vi "Martins HOT interface 120420.vi"() -> ()   [LabVIEW 2011] (continued)
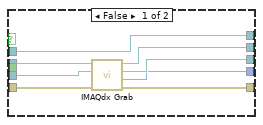
[diagram p6: hidden frame]
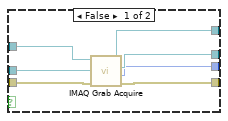
[diagram p7: hidden frame]
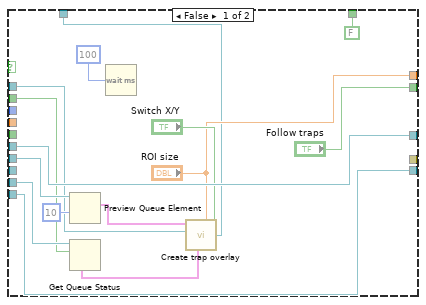
[diagram p9: hidden frame]
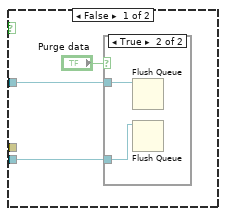
[diagram p11: hidden frame]
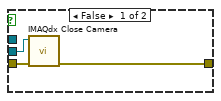
[diagram p16: hidden frame]
              tunnel: w260 -> [_ w344]
              tunnel: w254 -> [_ w343]
              tunnel: w259 -> [_ w342]
              tunnel: w258 -> [_ w341]
              tunnel: [w338 w339] -> w253
              tunnel: w252 -> [w338 w340]
              frame False {
              }
              frame True {
                n77 = call "compute path cluster.vi"("path queue"=w343, "Arrive simultaeously"=w341, "error in (no error)"=w340, "Step length\n(IMAQ pixels)"=w342, "waypoint queue"=w344) -> ("error out"=w339:errorcluster)  [unwired: 2 in]
              }
            }
            n78 = case "Follow path" shown="True" w255 {
              tunnel: w254 -> [_ w289]
              tunnel: w253 -> [_ w290]
              tunnel: w251 -> [_ w292]
              tunnel: w250 -> [_ w291]
              tunnel: w248 -> [_ w288]
              tunnel: w247 -> [w262 w269]
              tunnel: [w262 w268] -> w246
              tunnel: [w261 w263] -> w245
              tunnel: w244 -> [w261 _]
              frame False {
              }
              frame True {
                w283 = TRUE ("Visible")
                n79 = local write "Display path"(FALSE ("Display path")) -> ()
                n80 = Flush Queue "Flush Waypts"(queue=w291, error in (no error)=w290) -> (error out=w282:errorcluster)  [unwired: 2 out]
                n81 = Get Queue Status(queue=w289, error in (no error)=w282) -> (queue out=w286:refnum<queue>, error out=w281:errorcluster, # elements in queue=w285:i32)  [unwired: 1 in, 5 out]
                n82 = property on="Pause" class="Bool (strict)"(error in=w281, "Visible"=w283) -> (error out=w280:errorcluster)  [unwired: 1 in, 1 out]
                n83 = property on="cancel path" class="Bool"(error in=w280, "Visible"=w283) -> (error out=w279:errorcluster)  [unwired: 1 in, 1 out]
                n84 = for {
                  N: w285 -> [_]
                  tunnel: w279 -> [w311]
                  tunnel: w292 -> [w313]
                  tunnel: w286 -> [w309]
                  tunnel: [w309] -> w284
                  tunnel: [FALSE ("Group traps")] -> w264
                  shift-right: [w300] -> w263
                  shift-left: _ -> [w302]
                  tunnel: [w299] -> w278
                  tunnel: [w296] -> w276 mode=indexing
                  tunnel: [w297] -> w272
                  tunnel: [TRUE ("Display path")] -> w270
                  i -> [w297]
                  stop <- w306 stop-if-true
                  n85 = Dequeue Element(queue=w309, timeout in ms (-1)=0, error in (no error)=w311) -> (element=w301:T4, timed out?=w305:bool, error out=w312:errorcluster)  [unwired: 1 out]
                  n86 = while {
                    tunnel: [w330] -> w303
                    tunnel: ["cancel path"] -> w298
                    stop <- w332 stop-if-true
                    n87 = local read "Stop program"() -> (w330:bool)
                    n88 = Wait (ms)(milliseconds to wait="Step time \n(ms)") -> ()  [unwired: 1 out]
                    n89 = Or(x=w330, y="cancel path") -> (x .or. y?=w328:bool)
                    n90 = Implies(1:w328, 2:"Pause") -> (0:w332:bool)
                  }
                  n91 = case shown="True" "Skip step if \ntimed out" {
                    tunnel: w313 -> [w319 w324]
                    tunnel: w312 -> [w318 w322]
                    tunnel: [FALSE ("overflow?") w320] -> w304
                    tunnel: w301 -> [w317 w323]
                    tunnel: [w316 w321] -> w299
                    tunnel: 500 ("timeout in ms (-1)") -> [w315 _]
                    frame False {
                      n92 = Enqueue Element "Enqueue trap pos"(queue=w319, element=w317, timeout in ms (-1)=w315, error in (no error)=w318) -> (error out=w316:errorcluster)  [unwired: 2 out]
                    }
                    frame True {
                      n93 = Lossy Enqueue Element(queue=w324, element=w323, error in (no error)=w322) -> (overflow?=w320:bool, error out=w321:errorcluster)  [unwired: 2 out]
                    }
                  }
                  "Step skipped" <- w304
                  n94 = case shown="False" w303 {
                    tunnel: w302 -> [_ w326]
                    tunnel: w301 -> [w325 _]
                    tunnel: [w325 w326] -> w300
                    frame False {
                    }
                    frame True {
                    }
                  }
                  n95 = Or(x=w298, y=w303) -> (x .or. y?=w308:bool)
                  n96 = Or(x=w308, y=w305) -> (x .or. y?=w306:bool)
                  n97 = Tick Count (ms)() -> (millisecond timer value=w296:u32)
                }
                n98 = local read "Switch X/Y"() -> (w266:bool)
                n99 = call "Trap cluster 2 ROI.vi"("Switch X/Y"=w266, "Trap cluster"=w263, "ROI in"=w288) -> ("ROI out"=w287:T1)
                n100 = local write "Step skipped"(w264) -> ()
                n101 = local write "Display path"(w270) -> ()
                n102 = local write "Create path"(w264) -> ()
                n103 = local write "Group \nTraps"(w264) -> ()
                n104 = property on="Pause" class="Bool (strict)"(error in=w278, "Visible"=w264, "Value"=w264) -> (error out=w277:errorcluster)  [unwired: 1 in, 1 out]
                n105 = property on="cancel path" class="Bool"(error in=w277, "Visible"=w264) -> ()  [unwired: 1 in, 2 out]
                n106 = property on="follow path" class="Bool (strict)"("Value"=w264) -> ()  [unwired: 2 in, 2 out]
                n107 = property on="Image" class="ImageControl"(error in=w269, "ROI"=w287) -> (error out=w268:errorcluster)  [unwired: 1 in, 1 out]
                n108 = Array Max & Min(array=w276) -> (max value=w275:u32, min value=w274:u32)  [unwired: 2 out]
                n109 = Subtract(x=w275, y=w274) -> (x-y=w273:u32)
                n110 = Increment(x=w272) -> (x+1=w267:i32)
                n111 = Divide(x=w273, y=w267) -> (x/y=→"Average step time (ms)":dbl)
                n112 = Flush Queue "Flush Path"(queue=w284) -> ()  [unwired: 1 in, 3 out]
              }
            }
          }
        }
        n113 = case shown="True" "Apply Corrections" {
          frame False {
          }
          frame True {
            n114 = call "Apply Corrections.vi"() -> ()  [unwired: 1 in]
          }
        }
      }
      frame True {
        n115 = property on="Cancel calibration" class="Bool"("Visible"=w346) -> ()  [unwired: 2 in, 2 out]
        n116 = local read "Coordinate mapping \n(IMAQ to SLM)"() -> (w353:T6)
        n117 = flat-sequence {
          tunnel: [w369] -> w359
          tunnel: [w371] -> w358
          tunnel: w354 -> [w369]
          tunnel: w353 -> [w363]
          tunnel: [w360] -> w352
          tunnel: [w363] -> w351
          tunnel: w350 -> [w362]
          tunnel: [w361] -> w348
          tunnel: [w384] -> w357
          tunnel: w359 -> [w384]
          tunnel: w358 -> [w378]
          tunnel: [w380] -> w356
          tunnel: w355 -> [w383]
          tunnel: w352 -> [w382]
          tunnel: w351 -> [w379]
          tunnel: [w376] -> w349
          tunnel: w348 -> [w376]
          tunnel: w357 -> [w439]
          tunnel: w349 -> [w437]
          tunnel: [w436] -> w347
          frame #0 {
            w372 = u32 8 items=["Zoom Tool"=8, "Selection Tool"=0, "Pan Tool"=9, "Point Tool"=1, "Line Tool"=2, "Rectangle Tool"=3, "Rotated Rectangle Tool"=12, "Polyline Tool"=10, "Polygon Tool"=5, "Freehand Tool"=11, "Closed Freehand Tool"=6, "Ellipse Tool"=4, "Annulus Tool"=7] ("Current ROI Tool")
            n118 = Bundle By Name(cluster=w363, "sX"=0.0, "sY"=0.0, "cX"=1.0 ("sX"), "cY"=1.0) -> (w360:T6)
            n119 = local write "Coordinate mapping \n(IMAQ to SLM)"(w360) -> ()
            n120 = property on="ok" class="Bool"("Visible"=TRUE ("ROI Tool Buttons Visibile:Zoom Tool Button Visible")) -> ()  [unwired: 2 in, 2 out]
            n121 = property on="Image" class="ImageControl"("Current ROI Tool"=w372) -> ()  [unwired: 2 in, 2 out]
            n122 = Two Button Dialog(message="Mark the center of the \ndisplayed spot using the \nzoom and the point tool, \nthen click the OK button. \n(Will be repeated three times)", 1:"Cancel" ("F button name (\"Cancel\")"), 2:"Start calibration" ("T button name (\"OK\")")) -> (T button?=w371:bool)
            n123 = property on="Image" class="ImageControl"(error in=w362, "ROI"=T1 {"Global Rectangle"=[100, 100, 394, 354], "Contours"=[{"Contour Type"=0, "ROI Type"=1, "Points"=[100, 100]}]} ("ROI 2")) -> (error out=w361:errorcluster)  [unwired: 1 in, 1 out]
          }
          frame #1 {
            n124 = case shown="True" w378 {
              tunnel: w382 -> [w388 w399]
              tunnel: [w388 w394] -> w381
              tunnel: w383 -> [_ w390]
              tunnel: [TRUE ("Stop program") w389] -> w377
              frame False {
              }
              frame True {
                n125 = for {
                  tunnel: [w426] -> w408 mode=indexing
                  tunnel: [w425] -> w407 mode=indexing
                  tunnel: T4[] [{"X (IMAQ)"=[-64.0], "Y (IMAQ)"=[-64.0], "Z"=[0.0], "I"=[1.0], "Trap number"=[0], "ROI number"=[0], "Number of traps"=1, "Group"=[]}, {"X (IMAQ)"=[64.0], "Y (IMAQ)"=[-64.0], "Z"=[0.0], "I"=[1.0], "Trap number"=[0], "ROI number"=[0], "Number of traps"=1, "Group"=[]}, {"X (IMAQ)"=[-64.0], "Y (IMAQ)"=[64.0], "Z"=[0.0], "I"=[1.0], "Trap number"=[0], "ROI number"=[0], "Number of traps"=0, "Group"=[]}] -> [w423] mode=indexing
                  tunnel: [w420] -> w392 mode=indexing
                  tunnel: [w418] -> w391 mode=indexing
                  tunnel: w390 -> [w422]
                  tunnel: [w417] -> w389
                  stop <- w417 stop-if-true
                  n126 = while {
                    tunnel: [w433] -> w424
                    tunnel: [w429] -> w417
                    stop <- w431 stop-if-true
                    n127 = local read "Stop program"() -> (w430:bool)
                    n128 = Wait (ms)(milliseconds to wait=u32 50) -> ()  [unwired: 1 out]
                    n129 = Or(x=w430, y="Cancel calibration") -> (x .or. y?=w429:bool)
                    n130 = property on="Image" class="ImageControl"() -> ("ROI"=w433:T1)  [unwired: 2 in, 2 out]
                    n131 = Or(x="ok", y=w429) -> (x .or. y?=w431:bool)
                  }
                  n132 = Enqueue Element "Enqueue trap pos"(queue=w422, element=w423) -> ()  [unwired: 2 in, 3 out]
                  n133 = Unbundle By Name(w424) -> ("Global Rectangle"=w427:i32[])  [unwired: 1 out]
                  n134 = Unbundle By Name(w423) -> ("X (IMAQ)"=w421:sgl[], "Y (IMAQ)"=w419:sgl[])
                  n135 = Index Array(array=w421) -> (element=w420:sgl)  [unwired: 1 in]
                  n136 = Index Array(array=w419) -> (element=w418:sgl)  [unwired: 1 in]
                  n137 = Index Array(array=w427) -> (element #1=w426:i32, element #2=w425:i32)  [unwired: 2 in]
                }
                n138 = Index Array(array=w407) -> (element #1=w409:i32, element #2=w410:i32)  [unwired: 2 in]
                n139 = Index Array(array=w408) -> (element #1=w411:i32, element #2=w412:i32)  [unwired: 2 in]
                n140 = Subtract(x=w412, y=w411) -> (x-y=w404:i32)
                n141 = Subtract(x=w410, y=w409) -> (x-y=w402:i32)
                n142 = Absolute Value(x=w402) -> (abs(x)=w401:i32)
                n143 = Absolute Value(x=w404) -> (abs(x)=w403:i32)
                n144 = Less?(x=w403, y=w401) -> (x < y?=w400:bool)
                n145 = case shown="False" w400 {
                  tunnel: w408 -> [w414 w416]
                  tunnel: w407 -> [w413 w415]
                  tunnel: [w413 w416] -> w405
                  tunnel: [w414 w415] -> w406
                  frame False {
                  }
                  frame True {
                  }
                }
                n146 = formula code="cX = (xSLM[1] - xSLM[0]) / (xIMAQ[1] - xIMAQ[0]); \ncY = (ySLM[2] - ySLM[0]) / (yIMAQ[2] - yIMAQ[0]); \n\nsX = xSLM[0] - xIMAQ[0] *cX;\nsY = ySLM[0] - yIMAQ[0] *cY;"("xIMAQ"=w406, "yIMAQ"=w405, "xSLM"=w392, "ySLM"=w391) -> ("cX"=w398:dbl, "cY"=w397:dbl, "sX"=w396:dbl, "sY"=w395:dbl)
                n147 = property on="Switch X/Y" class="Bool (strict)"("Value"=w400) -> ()  [unwired: 2 in, 2 out]
                n148 = Bundle By Name(cluster=w399, "cX"=w398, "cY"=w397, "sX"=w396, "sY"=w395) -> (w394:T6)
              }
            }
            n149 = case "Calibration canceled?" shown="True" w377 {
              tunnel: w381 -> [w385 _]
              tunnel: [w385 w386] -> w380
              tunnel: w379 -> [_ w386]
              frame False {
              }
              frame True {
              }
            }
          }
          frame #2 {
            w435 = FALSE ("ROI Tool Buttons Visibile:Zoom Tool Button Visible")
            w438 = u32 1 items=["Zoom Tool"=8, "Selection Tool"=0, "Pan Tool"=9, "Point Tool"=1, "Line Tool"=2, "Rectangle Tool"=3, "Rotated Rectangle Tool"=12, "Polyline Tool"=10, "Polygon Tool"=5, "Freehand Tool"=11, "Closed Freehand Tool"=6, "Ellipse Tool"=4, "Annulus Tool"=7] ("Current ROI Tool")
            n150 = property on="Image" class="ImageControl"("Current ROI Tool"=w438, "Point Tool Button Visibile"=w435) -> ()  [unwired: 2 in, 2 out]
            n151 = property on="Image" class="ImageControl"(error in=w437, "ROI"=w439) -> (error out=w436:errorcluster)  [unwired: 1 in, 1 out]
            n152 = property on="Cancel" class="Bool"("Visible"=w435) -> ()  [unwired: 2 in, 2 out]
            n153 = property on="ok" class="Bool"("Visible"=w435) -> ()  [unwired: 2 in, 2 out]
          }
        }
        n154 = local write "Coordinate mapping \n(IMAQ to SLM)"(w356) -> ()
      }
    }
  }
  n155 = while "User input and events loop" {
    tunnel: w55 -> [w458]
    tunnel: w15 -> [w447]
    tunnel: w16 -> [w446]
    tunnel: w17 -> [w445]
    tunnel: [w444] -> w31
    tunnel: w30 -> [w443]
    tunnel: [w442] -> w29
    tunnel: w3 -> [w440]
    stop <- w450 stop-if-true
    w455 = u32 8 items=["Zoom Tool"=8, "Selection Tool"=0, "Pan Tool"=9, "Point Tool"=1, "Line Tool"=2, "Rectangle Tool"=3, "Rotated Rectangle Tool"=12, "Polyline Tool"=10, "Polygon Tool"=5, "Freehand Tool"=11, "Closed Freehand Tool"=6, "Ellipse Tool"=4, "Annulus Tool"=7] ("Current ROI Tool")
    w452 = T10 [enum."LCONTROL"] items=["0", "1", "2", "3", "4", "5", "6", "7", "8", "9", "A", "B", "C", "D", "E", "F", "G", "H", "I", "J", "K", "L", "M", "N", "O", "P", "Q", "R", "S", "T", "U", "V", "W", "X", "Y", "Z", "F1", "F2", "F3", "F4", "F5", "F6", "F7", "F8", "F9", "F10", "F11", "F12", "F13", "F14", "F15", "ADD", "BACK", "BACKSLASH", "CAPITAL", "COMMA", "DECIMAL", "DELETE", "DIVIDE", "DOWN", "END", "EQUALS", "ESCAPE", "GRAVE (`)", "HOME", "INSERT", "LBRACKET", "LCONTROL", "LEFT", "L ALT", "LSHIFT", "LWIN", "MINUS", "MULTIPLY", "NEXT", "NUMLOCK", "NUMPAD_0", "NUMPAD_1", "NUMPAD_2", "NUMPAD_3", "NUMPAD_4", "NUMPAD_5", "NUMPAD_6", "NUMPAD_7", "NUMPAD_8", "NUMPAD_9", "PAUSE", "PERIOD", "PRIOR (PG UP)", "RBRACKET", "RCONTROL", "RETURN", "RIGHT", "R ALT", "RSHIFT", "RWIN", "SCROLL", "SEMICOLON", "SLASH", "SPACE", "SUBTRACT", "TAB", "UP", "ENTER (num pad)", "' (quote)"] ("keys pressed")
    n156 = call-poly <vilib>:"Acquire Input Data.vi"("device ID"=w458, "error in (no error)"=w443) -> ("device ID"=w444:refnum<k1>, "keys pressed"=w451:T10, "error out"=w442:errorcluster)  [unwired: 15 out]
    n157 = property on="Image" class="ImageControl"() -> ("Current ROI Tool"=w454:u32)  [unwired: 2 in, 2 out]
    n158 = Equal?(x=w451, y=w452) -> (x = y?=w453:bool[])
    n159 = Not Equal?(x=w454, y=w455) -> (x != y?=w456:bool)
    n160 = Or Array Elements(Boolean array=w453) -> (logical OR=w457:bool)
    n161 = case shown="True" w456 {
      tunnel: w457 -> [_ w492]
      frame False {
      }
      frame True {
        n162 = case shown="False" w492 {
          frame False {
            w493 = u32 0 items=["Zoom Tool"=8, "Selection Tool"=0, "Pan Tool"=9, "Point Tool"=1, "Line Tool"=2, "Rectangle Tool"=3, "Rotated Rectangle Tool"=12, "Polyline Tool"=10, "Polygon Tool"=5, "Freehand Tool"=11, "Closed Freehand Tool"=6, "Ellipse Tool"=4, "Annulus Tool"=7] ("Current ROI Tool")
            n163 = property on="Image" class="ImageControl"("Current ROI Tool"=w493) -> ()  [unwired: 2 in, 2 out]
          }
          frame True {
            w494 = u32 1 items=["Zoom Tool"=8, "Selection Tool"=0, "Pan Tool"=9, "Point Tool"=1, "Line Tool"=2, "Rectangle Tool"=3, "Rotated Rectangle Tool"=12, "Polyline Tool"=10, "Polygon Tool"=5, "Freehand Tool"=11, "Closed Freehand Tool"=6, "Ellipse Tool"=4, "Annulus Tool"=7] ("Current ROI Tool")
            n164 = property on="Image" class="ImageControl"("Current ROI Tool"=w494) -> ()  [unwired: 2 in, 2 out]
          }
        }
      }
    }
    n165 = Wait (ms)(milliseconds to wait=u32 50) -> ()  [unwired: 1 out]
    n166 = case shown="False" "View Licence" {
      frame False {
      }
      frame True {
        n167 = call "View license.vi"() -> ()  [unwired: 1 in]
      }
    }
    n168 = event shown="[1] \"Display hologram\nand computed \nimage plane\": Value Change" {
      selector: _ -> [_ _ _ _ _ _ _ _ _]
      dyn-events: _ -> [_ _ _ _ _ _ _ _ _]
      timeout: 0 -> [_ _ _ _ _ _ _ _ _]
      tunnel: w447 -> [_ _ w469 _ _ _ _ _ _]
      tunnel: w446 -> [_ _ w468 _ _ _ _ _ _]
      tunnel: w445 -> [_ _ w472 _ _ _ _ _ _]
      tunnel: w440 -> [_ _ _ _ _ _ w484 _ _]
      event Timeout {
        n169 = event-data() -> ()  [unwired: 1 in, 2 out]
      }
      event "Display hologram\nand computed \nimage plane": Value Change {
        n170 = event-data() -> ("NewVal"=w460:bool)  [unwired: 1 in, 4 out]
        n171 = property on="Current trap pos" class="Clust (strict)"("Visible"=w460) -> ()  [unwired: 2 in, 2 out]
        n172 = property on="Displayed Hologram" class="IntGraph (strict)"("Visible"=w460) -> ()  [unwired: 2 in, 2 out]
        n173 = property on="Calculated image plane" class="IntGraph (strict)"("Visible"=w460) -> ()  [unwired: 2 in, 2 out]
        n174 = property on="Property Node" class="VI"() -> ("Front Panel.WinBounds"=w467:T11)  [unwired: 2 in, 2 out]
        n175 = Unbundle By Name(w467) -> ("right"=w466:i16, "left"=w465:i16)
        n176 = Subtract(x=w466, y=w465) -> (x-y=w464:i16)
        n177 = Select(t=i16 500 ("x-y"), s=w460, f=i16 196 ("x-y")) -> (s? t:f=w459:i16)
        n178 = Subtract(x=w464, y=w459) -> (x-y=w463:i16)
        n179 = property on="Splitter" class="Splitter"("Position"=w463) -> ()  [unwired: 2 in, 2 out]
      }
      event "Create path": Value Change {
        n180 = event-data() -> ()  [unwired: 1 in, 5 out]
        n181 = property on="follow path" class="Bool (strict)"("Value"=FALSE) -> ()  [unwired: 2 in, 2 out]
        n182 = Flush Queue "Flush path \nwaypt queue"(queue=w468) -> ()  [unwired: 1 in, 3 out]
        n183 = Preview Queue Element(queue=w469) -> (element=w470:T4, error out=w473:errorcluster)  [unwired: 2 in, 2 out]
        n184 = Flush Queue "Flush path queue"(queue=w472) -> (queue out=w471:refnum<queue>)  [unwired: 1 in, 2 out]
        n185 = Enqueue Element "Enqueue current \ntrap pos in path"(queue=w471, element=w470) -> ()  [unwired: 2 in, 3 out]
        n186 = Enqueue Element "Enqueue current \ntrap pos in path \nwaypts"(queue=w468, element=w470, error in (no error)=w473) -> ()  [unwired: 1 in, 3 out]
      }
      event "cancel path": Value Change {
        n187 = event-data() -> ()  [unwired: 1 in, 5 out]
        n188 = local write "Create path"(FALSE ("Visible")) -> ()
      }
      event "Image", "Group \nTraps", "Z", "I", "Coordinate mapping \n(IMAQ to SLM)": Mouse Down {
        w476 = FALSE ("Edit trap cluster")
        n189 = event-data() -> ()  [unwired: 1 in, 7 out]
        n190 = local write "Updating trap cluster"(TRUE ("Update trap positions")) -> ()
        n191 = local write "Edit trap cluster"(w476) -> ()
        n192 = call <vilib>:"Application Directory.vi"() -> ("Application Directory"=w477:path)
        n193 = Build Path(base path=w477, name or relative path="Sub VIs\\Edit trap cluster.vi") -> (appended path=w480:path)
        n194 = Open VI Reference(vi path=w480) -> (vi reference=w479:refnum<vi>)  [unwired: 5 in, 1 out]
        n195 = property class="VI"(reference=w479, "Front Panel.Open"=w476) -> ()  [unwired: 1 in, 2 out]
      }
      event "Group \nTraps", "Z", "I", "Image", "Coordinate mapping \n(IMAQ to SLM)": Mouse Up {
        n196 = event-data() -> ()  [unwired: 1 in, 7 out]
        n197 = flat-sequence {
          frame #0 {
            n198 = Wait (ms)(milliseconds to wait=u32 100) -> ()  [unwired: 1 out]
          }
          frame #1 {
            n199 = local write "Updating trap cluster"(FALSE ("Update trap positions")) -> ()
          }
        }
      }
      event "Video tracking": Value Change {
        n200 = event-data() -> ()  [unwired: 1 in, 5 out]
        n201 = for {
          tunnel: w484 -> [w485] mode=indexing
          n202 = call "IMAQ Clear Overlay"("Image"=w485) -> ()  [unwired: 9 in, 2 out]
        }
      }
      event "Display data": Value Change {
        n203 = event-data() -> ("NewVal"=w487:bool)  [unwired: 1 in, 4 out]
        n204 = call <vilib>:"Application Directory.vi"() -> ("Application Directory"=w486:path)
        n205 = Build Path(base path=w486, name or relative path="Sub VIs\\Display Cetroids (SubVI).vi") -> (appended path=w490:path)
        n206 = Open VI Reference(vi path=w490) -> (vi reference=w489:refnum<vi>)  [unwired: 5 in, 1 out]
        n207 = property class="VI"(reference=w489, "Front Panel.Open"=w487) -> ()  [unwired: 1 in, 2 out]
      }
      event "Edit trap cluster": Value Change {
        n208 = event-data() -> ("NewVal"=w491:bool)  [unwired: 1 in, 4 out]
        n209 = local write "Updating trap cluster"(w491) -> ()
      }
    }
    n210 = local read "Stop program"() -> (w450:bool)
  }
  n211 = disable-structure shown="Disabled" {
    disable-tunnel: [w511 _] -> w54
    disable-tunnel: [w510 _] -> w53
    disable-tunnel: w52 -> [w509 _]
    disable-tunnel: w50 -> [w508 _]
    disable-tunnel: w47 -> [w507 _]
    disable-tunnel: [w506 _] -> w45
    disable-tunnel: [w505 _] -> w44
    disable-tunnel: [w504 _] -> w43
    disable-tunnel: w22 -> [w503 _]
    disable-tunnel: w21 -> [w502 _]
    disable-tunnel: w20 -> [w501 _]
    disable-tunnel: w19 -> [w500 _]
    disable-tunnel: w18 -> [w499 _]
    disable-tunnel: w17 -> [w498 _]
    disable-tunnel: w15 -> [w497 _]
    disable-tunnel: w5 -> [w496 _]
    disable-tunnel: w4 -> [w495 _]
    frame Disabled {
      n212 = while "Image acquisition loop" {
        tunnel: w499 -> [w527]
        tunnel: w495 -> [w551]
        tunnel: w500 -> [w550]
        tunnel: [w523] -> w511
        tunnel: [w549] -> w510
        tunnel: w509 -> [w540]
        tunnel: w508 -> [w547]
        shift-right: [w546] -> _
        shift-left: _ -> [w545]
        tunnel: w507 -> [w544]
        shift-right: [w543] -> _
        shift-left: _ -> [w542]
        tunnel: [w540] -> w506
        tunnel: [w519] -> w505
        tunnel: [w539] -> w504
        tunnel: w503 -> [w538]
        tunnel: w501 -> [w537]
        tunnel: w497 -> [w536]
        tunnel: w498 -> [w535]
        tunnel: w502 -> [w533]
        tunnel: w496 -> [w522]
        i -> [w525]
        stop <- w548 stop-if-true
        n213 = case shown="True" w527 {
          tunnel: w551 -> [w577 w591]
          tunnel: w550 -> [w576 w590]
          tunnel: [w576 w589] -> w521
          tunnel: [w575 w588] -> w549
          tunnel: [w577 w587] -> w515
          tunnel: [w578 w586] -> w539
          tunnel: w538 -> [w578 w585]
          tunnel: w537 -> [_ w584]
          tunnel: w533 -> [w575 w583]
          tunnel: [_ w582] -> w532
          tunnel: w522 -> [_ w581]
          tunnel: w525 -> [_ w580]
          tunnel: "Video tracking" -> [_ w579]
          frame False {
          }
          frame True {
            n214 = case shown="True" w584 {
              tunnel: w591 -> [w599 w610]
              tunnel: [w597 w609] -> w589
              tunnel: [w596 w608] -> w588
              tunnel: w590 -> [w597 w607]
              tunnel: [w598 w606] -> w587
              tunnel: [w593 w605] -> w582
              tunnel: [w595 w604] -> w586
              tunnel: w585 -> [w594 w604]
              tunnel: w583 -> [w592 w603]
              tunnel: w581 -> [_ w602]
              tunnel: w580 -> [_ w601]
              tunnel: w579 -> [_ w600]
              frame False {
                n215 = call <vilib>:"IMAQdx Grab.vi"("error in"=w592, "Image In"=w599, "Session In"=w594) -> ("error out"=w596:errorcluster, "Buffer Number Out"=w593:u32, "Image Out"=w598:T2, "Session Out"=w595:T8)  [unwired: 5 in]
              }
              frame True {
                n216 = case shown="True" w602 {
                  tunnel: w610 -> [w617 _]
                  tunnel: [w616 w625] -> w609
                  tunnel: [w615 w627] -> w608
                  tunnel: w607 -> [w614 w622]
                  tunnel: [w613 w626] -> w606
                  tunnel: [w612 w624] -> w605
                  tunnel: w603 -> [w611 w623]
                  tunnel: w601 -> [_ w619]
                  tunnel: w600 -> [_ w618]
                  frame False {
                    n217 = call <vilib>:"IMAQ Grab Acquire.vi"("error in (no error)"=w611, "Image In"=w617, "IMAQ Session In"=w614) -> ("error out"=w615:errorcluster, "Acquired Buffer Number"=w612:u32, "Image Out"=w613:T2, "IMAQ Session Out"=w616:refnum<k11>)  [unwired: 1 in, 4 out]
                  }
                  frame True {
                    n218 = case shown="False" w618 {
                      tunnel: w623 -> [w631 w632]
                      tunnel: w622 -> [w630 _]
                      tunnel: [w629 w632] -> w621
                      tunnel: [w628 w633] -> w620
                      tunnel: w619 -> [_ w633]
                      frame False {
                        n219 = property class="IMAQ"(reference=w630, error in=w631) -> (error out=w629:errorcluster, "Last Valid Frame"=w628:u32)  [unwired: 1 out]
                      }
                      frame True {
                      }
                    }
                    n220 = call <vilib>:"IMAQ Extract Buffer.vi"("error in (no error)"=w621, "Buffer to extract"=w620, "IMAQ Session In"=w622) -> ("error out"=w627:errorcluster, "Buffer Number"=w624:i32, "Image Out"=w626:T2, "IMAQ Session Out"=w625:refnum<k11>)  [unwired: 3 in, 2 out]
                  }
                }
              }
            }
          }
        }
        n221 = case shown="True" "save image" {
          tunnel: w515 -> [w552 w557]
          tunnel: [w552 w556] -> w513
          frame False {
          }
          frame True {
            n222 = call "File Dialog"("start path"="start path") -> ("selected path"=w555:path, "cancelled"=w554:bool)  [unwired: 11 in, 2 out]
            n223 = case shown="False" w554 {
              tunnel: w557 -> [w560 w561]
              tunnel: [w559 w561] -> w556
              tunnel: w555 -> [w558 _]
              frame False {
                n224 = call-poly "IMAQ Write File 2"("File Path"=w558, "Image"=w560) -> ("Image Out (duplicate)"=w559:T2)  [unwired: 8 in, 1 out]
              }
              frame True {
              }
            }
          }
        }
        n225 = case shown="True" "threshold" {
          tunnel: w513 -> [w562 w569]
          tunnel: [w562 w567] -> w519
          frame False {
          }
          frame True {
            n226 = Unbundle By Name("Range") -> ("Lower value"=w564:sgl)
            n227 = Select(t=sgl 0.0 ("Lower value"), s="s", f=w564) -> (s? t:f=w566:sgl)
            n228 = Bundle By Name(cluster="Range", "Lower value"=w566) -> (w570:cluster{"Lower value":sgl, "Upper value":sgl})
            n229 = Select(t=w564, s="s", f=sgl 0.0) -> (s? t:f=w572:sgl)
            n230 = call "IMAQ Subtract"("Image Src A"=w569, "Constant"=w572) -> ("Image Dst Out"=w568:T2)  [unwired: 5 in, 1 out]
            n231 = call "IMAQ Threshold"("Keep/Replace Value (Replace)"=FALSE, "Range"=w570, "Image Src"=w568) -> ("Image Dst Out"=w567:T2)  [unwired: 7 in, 1 out]
          }
        }
        n232 = case shown="True" "Video tracking" {
          tunnel: w519 -> [w636 w651]
          tunnel: w540 -> [_ w664]
          tunnel: w547 -> [w648 w663]
          tunnel: w532 -> [_ w662]
          tunnel: [w648 w661] -> w531
          tunnel: [_ w660] -> w529
          tunnel: ["ROI size" w659] -> w546
          tunnel: w545 -> [_ w659]
          tunnel: w544 -> [w647 w658]
          tunnel: [w647 w657] -> w528
          tunnel: ["Follow traps" w656] -> w543
          tunnel: w542 -> [_ w656]
          tunnel: w535 -> [w641 _]
          tunnel: w536 -> [w640 w654]
          tunnel: "Display path" -> [w638 _]
          tunnel: [w635 w651] -> w518
          tunnel: [FALSE ("timed out?") w649] -> w516
          frame False {
            n233 = Preview Queue Element(queue=w640, timeout in ms (-1)=10) -> (element=w639:T4)  [unwired: 1 in, 3 out]
            n234 = Get Queue Status(queue=w641, return elements? (F)=w638) -> (elements=w642:T4[])  [unwired: 1 in, 7 out]
            n235 = Wait (ms)(milliseconds to wait=u32 100) -> ()  [unwired: 1 out]
            n236 = call "Create trap overlay.vi"("Current trap cluster"=w639, "Image in"=w636, "ROI size"="ROI size", "Switch X/Y"="Switch X/Y", "Path"=w642) -> ("Image Out"=w635:T2)
          }
          frame True {
            n237 = Preview Queue Element(queue=w654) -> (element=w655:T4)  [unwired: 2 in, 3 out]
            n238 = call "Position measurement.vi"("Image"=w651, "Trap positions"=w655, "ROIs"=w664, "Follow traps?"=w656, "Acquired Buffer Number"=w662, "ROI size"=w659) -> ("Position data out"=w653:T12)
            n239 = case shown="True" "Display data" {
              tunnel: w653 -> [_ w665]
              frame False {
              }
              frame True {
                n240 = call "Display Cetroids (SubVI).vi"("Measurement data"=w665) -> ()  [unwired: 8 in, 3 out]
              }
            }
            n241 = Enqueue Element(queue=w663, element=w653, timeout in ms (-1)=10000) -> (queue out=w661:refnum<queue>, timed out?=w649:bool, error out=w660:errorcluster)  [unwired: 1 in]
            n242 = Enqueue Element(queue=w658, element=w655) -> (queue out=w657:refnum<queue>)  [unwired: 2 in, 2 out]
          }
        }
        n243 = case shown="True" "?" {
          tunnel: w518 -> [_ w695]
          frame False {
          }
          frame True {
            "Image" <- w695
          }
        }
        n244 = call "IMAQ Quantify 2"("Image"=w513) -> ("Global Report"=→"Global Report":T3)  [unwired: 8 in, 2 out]
        n245 = Or(x="Save data", y=w516) -> (x .or. y?=w517:bool)
        n246 = case shown="True" w517 {
          tunnel: w531 -> [w667 w687]
          tunnel: w529 -> [_ w677]
          tunnel: w528 -> [w666 w676]
          frame False {
            n247 = case shown="True" "Purge data" {
              tunnel: w667 -> [_ w670]
              tunnel: w666 -> [_ w669]
              frame False {
              }
              frame True {
                n248 = Flush Queue(queue=w670) -> ()  [unwired: 1 in, 3 out]
                n249 = Flush Queue(queue=w669) -> ()  [unwired: 1 in, 3 out]
              }
            }
          }
          frame True {
            n250 = Flush Queue(queue=w687, error in (no error)=w677) -> (remaining elements=w683:T13)  [unwired: 2 out]
            n251 = Flush Queue(queue=w676, error in (no error)=w677) -> (remaining elements=w675:T4[])  [unwired: 2 out]
            n252 = for {
              tunnel: [w694] -> w686 mode=indexing
              tunnel: [w693] -> w685 mode=indexing
              tunnel: [w692] -> w678 mode=indexing
              tunnel: w683 -> [w691] mode=indexing
              tunnel: w675 -> [w690] mode=indexing
              tunnel: [w689] -> w674 mode=indexing
              tunnel: [w688] -> w673 mode=indexing
              workers-P: _ -> [_]
              n253 = Unbundle By Name(w691) -> ("Centroid X"=w694:dbl[], "Centroid Y"=w693:dbl[], "Acquired Buffer Number"=w692:u32)
              n254 = Unbundle By Name(w690) -> ("X (IMAQ)"=w689:sgl[], "Y (IMAQ)"=w688:sgl[])
            }
            n255 = Transpose 2D Array(2D array=w686) -> (transposed array=w681:dbl[][])
            n256 = Transpose 2D Array(2D array=w685) -> (transposed array=w680:dbl[][])
            n257 = Transpose 2D Array(2D array=w674) -> (transposed array=w672:sgl[][])
            n258 = Transpose 2D Array(2D array=w673) -> (transposed array=w671:sgl[][])
            n259 = Build Array (concatenate)(w678, w681, w680, w672, w671) -> (w682:dbl[][])
            n260 = Transpose 2D Array(2D array=w682) -> (transposed array=w679:dbl[][])
            n261 = call-poly <vilib>:"Write To Spreadsheet File.vi"("format (%.3f)"="%.9f", "2D data"=w679) -> ()  [unwired: 6 in, 1 out]
          }
        }
        n262 = property class="IMAQ"(reference=w521) -> (reference out=w523:refnum<k11>, "Lost Frames"=→"Lost Frames":u32)  [unwired: 1 in, 1 out]
        n263 = local read "Stop program"() -> (w548:bool)
      }
    }
    frame Enabled {
    }
  }
  n264 = property class="Bool (strict)"("Visible"=w42) -> ()  [unwired: 2 in, 2 out]
  n265 = property on="ROI size" class="DigNum (strict)"("Visible"=w42) -> ()  [unwired: 2 in, 2 out]
  n266 = property on="Video tracking" class="Bool (strict)"("Visible"=w42) -> ()  [unwired: 2 in, 2 out]
  n267 = property on="Save data" class="Bool"("Visible"=w42) -> ()  [unwired: 2 in, 2 out]
  n268 = property on="Follow traps" class="Bool (strict)"("Visible"=w42) -> ()  [unwired: 2 in, 2 out]
  n269 = property on="Purge data" class="Bool"("Visible"=w42) -> ()  [unwired: 2 in, 2 out]
  n270 = call "FreeGPUandSLM.vi"("error in"=w1) -> ("error out"=w33:errorcluster)  [unwired: 1 out]
  "CUDA/SLM error" <- w33
  n271 = call-poly <vilib>:"Close Input Device.vi"("error in (no error)"=w29, "device ID"=w31) -> ()  [unwired: 9 out]
  n272 = for {
    tunnel: w45 -> [w696] mode=indexing
    n273 = call "IMAQ Dispose"("Image"=w696) -> ()  [unwired: 5 in, 1 out]
  }
  n274 = case shown="True" w18 {
    tunnel: w54 -> [_ w702]
    tunnel: w53 -> [w697 w701]
    tunnel: w43 -> [_ w700]
    tunnel: w20 -> [_ w699]
    tunnel: [w697 w698] -> w35
    frame False {
    }
    frame True {
      n275 = case shown="True" w699 {
        tunnel: w702 -> [_ w708]
        tunnel: w701 -> [w705 w707]
        tunnel: [w704 w706] -> w698
        tunnel: w700 -> [w703 _]
        frame False {
          n276 = call <vilib>:"IMAQdx Close Camera.vi"("error in"=w705, "Session In"=w703) -> ("error out"=w704:errorcluster)  [unwired: 9 in]
        }
        frame True {
          n277 = call <vilib>:"IMAQ Close.vi"("error in (no error)"=w707, "IMAQ Session In"=w708) -> ("error out"=w706:errorcluster)  [unwired: 9 in]
        }
      }
    }
  }
  n278 = Merge Errors(w35, w34) -> (w32:errorcluster)
  "NI Vision error" <- w32
  n279 = call "IMAQ Dispose"("Image"=w44) -> ()  [unwired: 5 in, 1 out]
  n280 = Unbundle By Name(w36) -> ("Contours"=w41:T14)
  n281 = Index Array(array=w41) -> (element=w40:T15)  [unwired: 1 in]
  n282 = flat-sequence {
    tunnel: w33 -> [_]
    tunnel: w32 -> [_]
    frame #0 {
      n283 = local write "Stop program"(FALSE ("Stop program")) -> ()
    }
  }
  n284 = Unbundle By Name(w40) -> ("ROI Type"=w39:u32)
  n285 = Equal?(x=w39, y=u32 1) -> (x = y?=w37:bool)
  n286 = case shown="True" w37 {
    tunnel: w36 -> [_ w710]
    frame False {
    }
    frame True {
      n287 = local write "ROI"(w710) -> ()
    }
  }
